vi "CRYO_MASTER_FULL_dev.vi"() -> ()   [LabVIEW 2017] (continued)
              tunnel: [w493] -> w489
              tunnel: w491 -> [w508]
              tunnel: w489 -> [w496]
              tunnel: [w495] -> w488
              tunnel: w487 -> [w494]
              frame #0 {
                n241 = property class="TabCtl (strict)"("Val(Sgnl)"=T1."DMMs" ("Value (Signaling)")) -> ()  [unwired: 2 in, 2 out]
              }
              frame #1 {
                w506 = "_" ("string")
                n242 = local read "Cycle #"() -> (w504:u32)
                n243 = call "LV_UNIXTIME.vi"("current time"=w496) -> ("date/time string"=w507:string)  [unwired: 9 in, 1 out]
                n244 = Format Value(format string="%06d", value (0)=w504) -> (output string=w503:string)  [unwired: 1 in]
                n245 = Concatenate Strings(w494, w507, w506, w503, w506, "page6.png" ("string")) -> (w501:string)
                n246 = invoke class="TabCtl (strict)" method="Get Image"(error in=errorcluster {"status"=FALSE, "code"=0, "source"=""} ("error in (no error)")) -> (error out=w497:errorcluster, "image data"=w499:T23)  [unwired: 5 in, 4 out]
                n247 = Build Path(base path=w508, name or relative path=w501) -> (appended path=w500:path)
                n248 = call <vilib>:"Write PNG File.vi"("error in (no error)"=w497, "image data"=w499, "path to PNG file"=w500) -> ("error out"=w495:errorcluster)  [unwired: 7 in, 1 out]
              }
            }
            n249 = local write "error out (frontpanel screenshots)"(w488) -> ()
          }
          frame #6 {
            n250 = flat-sequence {
              tunnel: w512 -> [w515]
              tunnel: [w515] -> w511
              tunnel: w513 -> [w530]
              tunnel: w511 -> [w518]
              tunnel: [w517] -> w510
              tunnel: w509 -> [w516]
              frame #0 {
                n251 = property class="TabCtl (strict)"("Val(Sgnl)"=T1."DIAGRAM" ("Value (Signaling)")) -> ()  [unwired: 2 in, 2 out]
              }
              frame #1 {
                w528 = "_" ("string")
                n252 = local read "Cycle #"() -> (w526:u32)
                n253 = Format Value(format string="%06d", value (0)=w526) -> (output string=w525:string)  [unwired: 1 in]
                n254 = call "LV_UNIXTIME.vi"("current time"=w518) -> ("date/time string"=w529:string)  [unwired: 9 in, 1 out]
                n255 = Concatenate Strings(w516, w529, w528, w525, w528, "page7.png" ("string")) -> (w523:string)
                n256 = invoke class="TabCtl (strict)" method="Get Image"(error in=errorcluster {"status"=FALSE, "code"=0, "source"=""} ("error in (no error)")) -> (error out=w519:errorcluster, "image data"=w521:T23)  [unwired: 5 in, 4 out]
                n257 = Build Path(base path=w530, name or relative path=w523) -> (appended path=w522:path)
                n258 = call <vilib>:"Write PNG File.vi"("error in (no error)"=w519, "image data"=w521, "path to PNG file"=w522) -> ("error out"=w517:errorcluster)  [unwired: 7 in, 1 out]
              }
            }
            n259 = local write "error out (frontpanel screenshots)"(w510) -> ()
          }
          frame #7 {
            n260 = flat-sequence {
              tunnel: w534 -> [w537]
              tunnel: [w537] -> w533
              tunnel: w535 -> [w552]
              tunnel: w533 -> [w540]
              tunnel: [w539] -> w532
              tunnel: w531 -> [w538]
              frame #0 {
                n261 = property class="TabCtl (strict)"("Val(Sgnl)"=T1."CHF" ("Value (Signaling)")) -> ()  [unwired: 2 in, 2 out]
              }
              frame #1 {
                w550 = "_" ("string")
                n262 = local read "Cycle #"() -> (w548:u32)
                n263 = Format Value(format string="%06d", value (0)=w548) -> (output string=w547:string)  [unwired: 1 in]
                n264 = call "LV_UNIXTIME.vi"("current time"=w540) -> ("date/time string"=w551:string)  [unwired: 9 in, 1 out]
                n265 = Concatenate Strings(w538, w551, w550, w547, w550, "page8.png" ("string")) -> (w545:string)
                n266 = invoke class="TabCtl (strict)" method="Get Image"(error in=errorcluster {"status"=FALSE, "code"=0, "source"=""} ("error in (no error)")) -> (error out=w541:errorcluster, "image data"=w543:T23)  [unwired: 5 in, 4 out]
                n267 = Build Path(base path=w552, name or relative path=w545) -> (appended path=w544:path)
                n268 = call <vilib>:"Write PNG File.vi"("error in (no error)"=w541, "image data"=w543, "path to PNG file"=w544) -> ("error out"=w539:errorcluster)  [unwired: 7 in, 1 out]
              }
            }
            n269 = local write "error out (frontpanel screenshots)"(w532) -> ()
          }
          frame #8 {
            n270 = flat-sequence {
              tunnel: w556 -> [w559]
              tunnel: [w559] -> w555
              tunnel: w557 -> [w574]
              tunnel: w555 -> [w562]
              tunnel: [w561] -> w554
              tunnel: w553 -> [w560]
              frame #0 {
                n271 = property class="TabCtl (strict)"("Val(Sgnl)"=T1."(Plc. hld.)" ("Value (Signaling)")) -> ()  [unwired: 2 in, 2 out]
              }
              frame #1 {
                w572 = "_" ("string")
                n272 = local read "Cycle #"() -> (w570:u32)
                n273 = Format Value(format string="%06d", value (0)=w570) -> (output string=w569:string)  [unwired: 1 in]
                n274 = call "LV_UNIXTIME.vi"("current time"=w562) -> ("date/time string"=w573:string)  [unwired: 9 in, 1 out]
                n275 = Concatenate Strings(w560, w573, w572, w569, w572, "page8.png" ("string")) -> (w567:string)
                n276 = invoke class="TabCtl (strict)" method="Get Image"(error in=errorcluster {"status"=FALSE, "code"=0, "source"=""} ("error in (no error)")) -> (error out=w563:errorcluster, "image data"=w565:T23)  [unwired: 5 in, 4 out]
                n277 = Build Path(base path=w574, name or relative path=w567) -> (appended path=w566:path)
                n278 = call <vilib>:"Write PNG File.vi"("error in (no error)"=w563, "image data"=w565, "path to PNG file"=w566) -> ("error out"=w561:errorcluster)  [unwired: 7 in, 1 out]
              }
            }
            n279 = local write "error out (frontpanel screenshots)"(w554) -> ()
          }
          frame #9 {
            n280 = local write "Frontpanel screenshots"(FALSE ("Frontpanel screenshots")) -> ()
          }
        }
        "error out (frontpanel screenshots)" <- w373
        n281 = property class="TabCtl (strict)"("Val(Sgnl)"=w371) -> ()  [unwired: 2 in, 2 out]
      }
      event "Stop Button": Value Change {
        n282 = event-data() -> ()  [unwired: 1 in, 3 out]
      }
    }
    n283 = Wait (ms)(milliseconds to wait=u32 123) -> ()  [unwired: 1 out]
  }
  n284 = while {
    stop <- w581 stop-if-true
    n285 = event shown="[5] \"Plot selecter LSI218(1)     1      2     3     4\", \"Plot selecter LSI218(2)     1      2     3     4\", \"Plot selecter (USB6210)     1      2     3     4\", \"Plot selecter LSI336       1      2     3     4\", \"Plot selecter (USB6218)     1      2     3     4\": Value Change" {
      selector: _ -> [_ _ _ _ _ _ _ _ _ _ _]
      dyn-events: _ -> [_ _ _ _ _ _ _ _ _ _ _]
      timeout: _ -> [_ _ _ _ _ _ _ _ _ _ _]
      tunnel: [_ _ _ _ _ _ _ _ _ _ TRUE] -> w581
      tunnel: [errorcluster {"status"=FALSE, "code"=0, "source"=""} ("error out") w585 _ _ _ _ w721 w738 w755 w772 errorcluster {"status"=FALSE, "code"=0, "source"=""} ("error out")] -> w577
      event Timeout {
        n286 = event-data() -> ()  [unwired: 1 in, 3 out]
      }
      event "log/linear 1": Value Change {
        n287 = event-data() -> ()  [unwired: 1 in, 6 out]
        n288 = flat-sequence {
          tunnel: [w586] -> w585
          frame #0 {
            n289 = Boolean To (0,1)(Boolean="log/linear 1") -> (0, 1=w591:i16)
            n290 = control-ref of="Graph 1"() -> (w587:refnum<vi>)
            n291 = property class="XYGraph (strict)"(reference=w587, error in=errorcluster {"status"=FALSE, "code"=0, "source"=""} ("error in (no error)"), "YScale.Mapping Mode"=w591) -> (error out=w589:errorcluster)  [unwired: 1 out]
            n292 = control-ref of="error out (USB6210)"() -> (w590:refnum<vi>)
            n293 = property class="Clust (strict)"(reference=w590, "Val(Sgnl)"=w589) -> (error out=w586:errorcluster)  [unwired: 1 in, 1 out]
          }
        }
      }
      event "log/linear 2": Value Change {
        n294 = event-data() -> ()  [unwired: 1 in, 6 out]
        n295 = flat-sequence {
          frame #0 {
            n296 = Boolean To (0,1)(Boolean="log/linear 2") -> (0, 1=w597:i16)
            n297 = control-ref of="Graph 2"() -> (w595:refnum<vi>)
            n298 = property class="XYGraph (strict)"(reference=w595, error in=errorcluster {"status"=FALSE, "code"=0, "source"=""} ("error in (no error)"), "YScale.Mapping Mode"=w597) -> (error out=w596:errorcluster)  [unwired: 1 out]
            n299 = control-ref of="error out (USB6210)"() -> (w594:refnum<vi>)
            n300 = property class="Clust (strict)"(reference=w594, "Value"=w596) -> ()  [unwired: 1 in, 2 out]
          }
        }
      }
      event "log/linear 3": Value Change {
        n301 = event-data() -> ()  [unwired: 1 in, 6 out]
        n302 = flat-sequence {
          frame #0 {
            n303 = Boolean To (0,1)(Boolean="log/linear 3") -> (0, 1=w603:i16)
            n304 = control-ref of="Graph 3"() -> (w599:refnum<vi>)
            n305 = property class="XYGraph (strict)"(reference=w599, error in=errorcluster {"status"=FALSE, "code"=0, "source"=""} ("error in (no error)"), "YScale.Mapping Mode"=w603) -> (error out=w602:errorcluster)  [unwired: 1 out]
            n306 = control-ref of="error out (USB6210)"() -> (w601:refnum<vi>)
            n307 = property class="Clust (strict)"(reference=w601, "Value"=w602) -> ()  [unwired: 1 in, 2 out]
          }
        }
      }
      event "log/linear 4": Value Change {
        n308 = event-data() -> ()  [unwired: 1 in, 6 out]
        n309 = flat-sequence {
          frame #0 {
            n310 = Boolean To (0,1)(Boolean="log/linear 4") -> (0, 1=w609:i16)
            n311 = control-ref of="Graph 4"() -> (w605:refnum<vi>)
            n312 = property class="XYGraph (strict)"(reference=w605, error in=errorcluster {"status"=FALSE, "code"=0, "source"=""} ("error in (no error)"), "YScale.Mapping Mode"=w609) -> (error out=w608:errorcluster)  [unwired: 1 out]
            n313 = control-ref of="error out (USB6210)"() -> (w607:refnum<vi>)
            n314 = property class="Clust (strict)"(reference=w607, "Value"=w608) -> ()  [unwired: 1 in, 2 out]
          }
        }
      }
      event "Plot selecter LSI218(1)\n    1      2     3     4", "Plot selecter LSI218(2)\n    1      2     3     4", "Plot selecter (USB6210)\n    1      2     3     4", "Plot selecter LSI336 \n     1      2     3     4", "Plot selecter (USB6218)\n    1      2     3     4": Value Change {
        n315 = event-data() -> ()  [unwired: 1 in, 6 out]
        n316 = local read "Labels (HP34401 LM)"() -> (w616:string[])
        n317 = call "BuildPlotLegends.vi"("Plot selecter \n    1      2     3     4"="Plot selecter (HP34401A)\n    1      2     3     4", "AllLabels"=w616) -> ("Series 4"=w611:string[], "Series 3"=w612:string[], "Series 2"=w613:string[], "Series 1"=w614:string[])  [unwired: 6 in]
        n318 = local read "All Labels (USB6210)"() -> (w633:string[])
        n319 = local read "All Labels (USB6218)"() -> (w622:string[])
        n320 = local read "Labels LSI218 (1)"() -> (w635:string[])
        n321 = local read "Labels LSI218 (2)"() -> (w636:string[])
        n322 = local read "Labels LSI336"() -> (w628:string[])
        n323 = call "BuildPlotLegends_LSI218.vi"("Plot selecter (2)\n    1      2     3     5"="Plot selecter LSI218(2)\n    1      2     3     4", "Plot selecter (1)\n    1      2     3     4"="Plot selecter LSI218(1)\n    1      2     3     4", "Labels (2)"=w636, "Labels (1)"=w635) -> ("Series 4"=w646:string[], "Series 3"=w644:string[], "Series 2"=w642:string[], "Series 1"=w640:string[])  [unwired: 4 in]
        n324 = call "BuildPlotLegends.vi"("Plot selecter \n    1      2     3     4"="Plot selecter (USB6210)\n    1      2     3     4", "AllLabels"=w633) -> ("Series 4"=w645:string[], "Series 3"=w643:string[], "Series 2"=w641:string[], "Series 1"=w639:string[])  [unwired: 6 in]
        n325 = call "BuildPlotLegends.vi"("Plot selecter \n    1      2     3     4"="Plot selecter LSI336 \n     1      2     3     4", "AllLabels"=w628) -> ("Series 4"=w623:string[], "Series 3"=w624:string[], "Series 2"=w625:string[], "Series 1"=w626:string[])  [unwired: 6 in]
        n326 = call "BuildPlotLegends.vi"("Plot selecter \n    1      2     3     4"="Plot selecter (USB6218)\n    1      2     3     4", "AllLabels"=w622) -> ("Series 4"=w618:string[], "Series 3"=w617:string[], "Series 2"=w619:string[], "Series 1"=w620:string[])  [unwired: 6 in]
        n327 = Build Array (concatenate)(w641, w642, w625, w619, w613) -> (w630:string[])
        "Series 2" <- w630
        n328 = Build Array (concatenate)(w643, w644, w624, w617, w612) -> (w631:string[])
        "Series 3" <- w631
        n329 = Build Array (concatenate)(w645, w646, w623, w618, w611) -> (w632:string[])
        "Series 4" <- w632
        n330 = Build Array (concatenate)(w639, w640, w626, w620, w614) -> (w629:string[])
        "Series 1" <- w629
        n331 = stacked-sequence {
          tunnel: [w656 _ _ _] -> w650
          tunnel: [_ w674 _ _] -> w651
          tunnel: [_ _ w691 _] -> w649
          tunnel: [_ _ _ w708] -> w648
          tunnel: w629 -> [w654 _ _ _]
          tunnel: w630 -> [_ w672 _ _]
          tunnel: w631 -> [_ _ w689 _]
          tunnel: w632 -> [_ _ _ w706]
          frame #0 {
            n332 = Array Size(array=w654) -> (size(s)=w658:i32)
            n333 = control-ref of="Graph 1"() -> (w652:refnum<vi>)
            n334 = property class="XYGraph (strict)"(reference=w652) -> ("LegNumRows"=w653:u32)  [unwired: 1 in, 2 out]
            n335 = for {
              N: w653 -> [_]
              tunnel: w652 -> [w667]
              shift-right: [w665] -> w657
              shift-left: errorcluster {"status"=FALSE, "code"=0, "source"=""} ("error in (no error)") -> [w666]
              i -> [w669]
              n336 = property class="XYGraph (strict)"(reference=w667, error in=w666, "Active Plot"=w669, "Plot.Plot Name"="") -> (error out=w665:errorcluster)  [unwired: 1 out]
            }
            n337 = for {
              N: w658 -> [_]
              tunnel: w652 -> [w663]
              shift-right: [w661] -> w656
              shift-left: w657 -> [w662]
              tunnel: w654 -> [w660] mode=indexing
              i -> [w664]
              n338 = property class="XYGraph (strict)"(reference=w663, error in=w662, "Active Plot"=w664, "Plot.Plot Name"=w660, "Plot.Visible?"=TRUE ("Plot.Visible")) -> (error out=w661:errorcluster)  [unwired: 1 out]
            }
          }
          frame #1 {
            n339 = Array Size(array=w672) -> (size(s)=w676:i32)
            n340 = control-ref of="Graph 2"() -> (w671:refnum<vi>)
            n341 = property class="XYGraph (strict)"(reference=w671) -> ("LegNumRows"=w670:u32)  [unwired: 1 in, 2 out]
            n342 = for {
              N: w670 -> [_]
              shift-right: [w683] -> w675
              shift-left: errorcluster {"status"=FALSE, "code"=0, "source"=""} ("error in (no error)") -> [w684]
              tunnel: w671 -> [w682]
              i -> [w686]
              n343 = property class="XYGraph (strict)"(reference=w682, error in=w684, "Active Plot"=w686, "Plot.Plot Name"="") -> (error out=w683:errorcluster)  [unwired: 1 out]
            }
            n344 = for {
              N: w676 -> [_]
              shift-right: [w679] -> w674
              shift-left: w675 -> [w680]
              tunnel: w672 -> [w678] mode=indexing
              tunnel: w671 -> [w677]
              i -> [w681]
              n345 = property class="XYGraph (strict)"(reference=w677, error in=w680, "Active Plot"=w681, "Plot.Plot Name"=w678) -> (error out=w679:errorcluster)  [unwired: 1 out]
            }
          }
          frame #2 {
            n346 = Array Size(array=w689) -> (size(s)=w693:i32)
            n347 = control-ref of="Graph 3"() -> (w687:refnum<vi>)
            n348 = property class="XYGraph (strict)"(reference=w687) -> ("LegNumRows"=w688:u32)  [unwired: 1 in, 2 out]
            n349 = for {
              N: w688 -> [_]
              tunnel: w687 -> [w701]
              shift-right: [w699] -> w692
              shift-left: errorcluster {"status"=FALSE, "code"=0, "source"=""} ("error in (no error)") -> [w700]
              i -> [w703]
              n350 = property class="XYGraph (strict)"(reference=w701, error in=w700, "Active Plot"=w703, "Plot.Plot Name"="") -> (error out=w699:errorcluster)  [unwired: 1 out]
            }
            n351 = for {
              N: w693 -> [_]
              tunnel: w687 -> [w697]
              shift-right: [w695] -> w691
              shift-left: w692 -> [w696]
              tunnel: w689 -> [w694] mode=indexing
              i -> [w698]
              n352 = property class="XYGraph (strict)"(reference=w697, error in=w696, "Active Plot"=w698, "Plot.Plot Name"=w694) -> (error out=w695:errorcluster)  [unwired: 1 out]
            }
          }
          frame #3 {
            n353 = Array Size(array=w706) -> (size(s)=w710:i32)
            n354 = control-ref of="Graph 4"() -> (w704:refnum<vi>)
            n355 = property class="XYGraph (strict)"(reference=w704) -> ("LegNumRows"=w705:u32)  [unwired: 1 in, 2 out]
            n356 = for {
              N: w705 -> [_]
              tunnel: w704 -> [w718]
              shift-right: [w716] -> w709
              shift-left: errorcluster {"status"=FALSE, "code"=0, "source"=""} ("error in (no error)") -> [w717]
              i -> [w720]
              n357 = property class="XYGraph (strict)"(reference=w718, error in=w717, "Active Plot"=w720, "Plot.Plot Name"="") -> (error out=w716:errorcluster)  [unwired: 1 out]
            }
            n358 = for {
              N: w710 -> [_]
              tunnel: w704 -> [w714]
              shift-right: [w712] -> w708
              shift-left: w709 -> [w713]
              tunnel: w706 -> [w711] mode=indexing
              i -> [w715]
              n359 = property class="XYGraph (strict)"(reference=w714, error in=w713, "Active Plot"=w715, "Plot.Plot Name"=w711) -> (error out=w712:errorcluster)  [unwired: 1 out]
            }
          }
        }
        n360 = Merge Errors(w650, w651, w649, w648) -> (→"Plot errors":errorcluster)
      }
      event "Take Screenshot! 1": Value Change {
        n361 = event-data() -> ()  [unwired: 1 in, 6 out]
        n362 = flat-sequence {
          tunnel: [w722] -> w721
          frame #0 {
            n363 = flat-sequence {
              tunnel: [w723] -> w722
              frame #0 {
                w732 = "_" ("string")
                n364 = Get Date/Time In Seconds() -> (seconds since 1Jan1904=w729:timestamp)
                n365 = local read "RUN Identifier"() -> (w734:string)
                n366 = call "LV_UNIXTIME.vi"("current time"=w729) -> ("date/time string"=w733:string)  [unwired: 9 in, 1 out]
                n367 = control-ref of="Graph 1"() -> (w728:refnum<vi>)
                n368 = Concatenate Strings(w734, w732, w733, w732, "FIle suffix 1", ".png" ("string")) -> (w736:string)
                n369 = local read "Base Path"() -> (w735:path)
                n370 = invoke class="XYGraph (strict)" method="Get Image"(reference=w728, error in=errorcluster {"status"=FALSE, "code"=0, "source"=""} ("error in (no error)")) -> (error out=w724:errorcluster, "image data"=w727:T23)  [unwired: 4 in, 4 out]
                n371 = Build Path(base path=w735, name or relative path=w736) -> (appended path=w726:path)
                n372 = call <vilib>:"Write PNG File.vi"("error in (no error)"=w724, "image data"=w727, "path to PNG file"=w726) -> ("error out"=w723:errorcluster)  [unwired: 7 in, 1 out]
              }
              frame #1 {
                n373 = local write "Take Screenshot! 1"(FALSE ("Take Screenshot! 1")) -> ()
              }
            }
          }
        }
      }
      event "Take Screenshot! 2": Value Change {
        n374 = event-data() -> ()  [unwired: 1 in, 6 out]
        n375 = flat-sequence {
          tunnel: [w739] -> w738
          frame #0 {
            n376 = flat-sequence {
              tunnel: [w745] -> w739
              frame #0 {
                w749 = "_" ("string")
                n377 = Get Date/Time In Seconds() -> (seconds since 1Jan1904=w746:timestamp)
                n378 = local read "RUN Identifier"() -> (w751:string)
                n379 = call "LV_UNIXTIME.vi"("current time"=w746) -> ("date/time string"=w750:string)  [unwired: 9 in, 1 out]
                n380 = control-ref of="Graph 2"() -> (w740:refnum<vi>)
                n381 = Concatenate Strings(w751, w749, w750, w749, "FIle suffix 2", ".png" ("string")) -> (w753:string)
                n382 = local read "Base Path"() -> (w752:path)
                n383 = invoke class="XYGraph (strict)" method="Get Image"(reference=w740, error in=errorcluster {"status"=FALSE, "code"=0, "source"=""} ("error in (no error)")) -> (error out=w744:errorcluster, "image data"=w742:T23)  [unwired: 4 in, 4 out]
                n384 = Build Path(base path=w752, name or relative path=w753) -> (appended path=w741:path)
                n385 = call <vilib>:"Write PNG File.vi"("error in (no error)"=w744, "image data"=w742, "path to PNG file"=w741) -> ("error out"=w745:errorcluster)  [unwired: 7 in, 1 out]
              }
              frame #1 {
                n386 = local write "Take Screenshot! 2"(FALSE ("Take Screenshot! 1")) -> ()
              }
            }
          }
        }
      }
      event "Take Screenshot! 3": Value Change {
        n387 = event-data() -> ()  [unwired: 1 in, 6 out]
        n388 = flat-sequence {
          tunnel: [w756] -> w755
          frame #0 {
            n389 = flat-sequence {
              tunnel: [w758] -> w756
              frame #0 {
                w766 = "_" ("string")
                n390 = Get Date/Time In Seconds() -> (seconds since 1Jan1904=w764:timestamp)
                n391 = local read "RUN Identifier"() -> (w768:string)
                n392 = call "LV_UNIXTIME.vi"("current time"=w764) -> ("date/time string"=w767:string)  [unwired: 9 in, 1 out]
                n393 = control-ref of="Graph 3"() -> (w761:refnum<vi>)
                n394 = Concatenate Strings(w768, w766, w767, w766, "FIle suffix 3", ".png" ("string")) -> (w770:string)
                n395 = local read "Base Path"() -> (w769:path)
                n396 = invoke class="XYGraph (strict)" method="Get Image"(reference=w761, error in=errorcluster {"status"=FALSE, "code"=0, "source"=""} ("error in (no error)")) -> (error out=w759:errorcluster, "image data"=w757:T23)  [unwired: 4 in, 4 out]
                n397 = Build Path(base path=w769, name or relative path=w770) -> (appended path=w762:path)
                n398 = call <vilib>:"Write PNG File.vi"("error in (no error)"=w759, "image data"=w757, "path to PNG file"=w762) -> ("error out"=w758:errorcluster)  [unwired: 7 in, 1 out]
              }
              frame #1 {
                n399 = local write "Take Screenshot! 3"(FALSE ("Take Screenshot! 1")) -> ()
              }
            }
          }
        }
      }
      event "Take Screenshot! 4": Value Change {
        n400 = event-data() -> ()  [unwired: 1 in, 6 out]
        n401 = flat-sequence {
          tunnel: [w773] -> w772
          frame #0 {
            n402 = flat-sequence {
              tunnel: [w776] -> w773
              frame #0 {
                w783 = "_" ("string")
                n403 = Get Date/Time In Seconds() -> (seconds since 1Jan1904=w781:timestamp)
                n404 = local read "RUN Identifier"() -> (w785:string)
                n405 = call "LV_UNIXTIME.vi"("current time"=w781) -> ("date/time string"=w784:string)  [unwired: 9 in, 1 out]
                n406 = control-ref of="Graph 4"() -> (w777:refnum<vi>)
                n407 = Concatenate Strings(w785, w783, w784, w783, "FIle suffix 4", ".png" ("string")) -> (w787:string)
                n408 = local read "Base Path"() -> (w786:path)
                n409 = invoke class="XYGraph (strict)" method="Get Image"(reference=w777, error in=errorcluster {"status"=FALSE, "code"=0, "source"=""} ("error in (no error)")) -> (error out=w774:errorcluster, "image data"=w778:T23)  [unwired: 4 in, 4 out]
                n410 = Build Path(base path=w786, name or relative path=w787) -> (appended path=w779:path)
                n411 = call <vilib>:"Write PNG File.vi"("error in (no error)"=w774, "image data"=w778, "path to PNG file"=w779) -> ("error out"=w776:errorcluster)  [unwired: 7 in, 1 out]
              }
              frame #1 {
                n412 = local write "Take Screenshot! 4"(FALSE ("Take Screenshot! 1")) -> ()
              }
            }
          }
        }
      }
      event "Stop Button": Value Change {
        n413 = event-data() -> ()  [unwired: 1 in, 6 out]
      }
    }
    "error out (graph operations)" <- w577
    n414 = local write "Take Screenshot! 1"(FALSE ("Take Screenshot! 1")) -> ()
    n415 = local write "Take Screenshot! 2"(FALSE ("Take Screenshot! 1")) -> ()
    n416 = Wait (ms)(milliseconds to wait=u32 1000) -> ()  [unwired: 1 out]
    n417 = local write "Take Screenshot! 3"(FALSE ("Take Screenshot! 1")) -> ()
    n418 = local write "Take Screenshot! 4"(FALSE ("Take Screenshot! 1")) -> ()
  }
  n419 = while {
    i -> [w795]
    stop <- w792 stop-if-true
    n420 = Equal?(x=w795, y=0) -> (x = y?=w793:bool)
    n421 = case shown="True" w793 {
      frame False {
      }
      frame True {
        n422 = property on="Agilent\nIntialized?" class="Bool (strict)"("Val(Sgnl)"=FALSE ("Value (Signaling)")) -> ()  [unwired: 2 in, 2 out]
      }
    }
    n423 = Wait (ms)(milliseconds to wait=u32 123) -> ()  [unwired: 1 out]
    n424 = event shown="[4] \"V_lim_up (V)\", \"V_lim_low (V)\": Value Change" {
      selector: _ -> [_ _ _ _ _]
      dyn-events: _ -> [_ _ _ _ _]
      timeout: _ -> [_ _ _ _ _]
      tunnel: [FALSE ("Value (Signaling)") TRUE ("Value (Signaling)") _ _ _] -> w792
      tunnel: "VISA (Agilent 34402)" -> [_ _ w801 w804 _]
      event Timeout {
        n425 = event-data() -> ()  [unwired: 1 in, 3 out]
      }
      event "Stop Button": Value Change {
        n426 = event-data() -> ()  [unwired: 1 in, 3 out]
      }
      event "Initialize (Agilent)": Value Change {
        n427 = event-data() -> ()  [unwired: 1 in, 3 out]
        n428 = property on="Agilent\nIntialized?" class="Bool (strict)"("Val(Sgnl)"=TRUE ("Value (Signaling)")) -> ()  [unwired: 2 in, 2 out]
        n429 = call "Initialize.vi"("error in (no error)"=errorcluster {"status"=FALSE, "code"=0, "source"=""}, "VISA resource name"=w801) -> ("error out"=→"error out (Agilent)":errorcluster)  [unwired: 8 in, 1 out]
      }
      event "OUTPUT \nKenwood", "Kenwood set V (V)": Value Change {
        n430 = local read "Agilent\nIntialized?"() -> (w803:bool)
        n431 = event-data() -> ()  [unwired: 1 in, 3 out]
        n432 = case shown="True" w803 {
          tunnel: w804 -> [_ w810]
          frame False {
          }
          frame True {
            w812 = u16 0 items=["DC", "Sine", "Square", "Triangle", "Ramp", "Pulse", "Noise", "Sinc", "Negative Ramp", "Exponential Rise", "Exponential Fall", "Cardiac"] ("Waveform Function (1: Sine)")
            n433 = xnode "Formula"("X1"="Kenwood set V (V)") -> ("Result"=w805:dbl)  [unwired: 1 in, 1 out]
            n434 = call "Configure Standard Waveform.vi"("DC Offset (0.00 V)"=w805, "Frequency (1000 Hz)"=1.0, "error in (no error)"=errorcluster {"status"=FALSE, "code"=0, "source"=""}, "Amplitude (1)"=1.0, "Waveform Function (1: Sine)"=w812, "VISA resource name"=w810) -> ("error out"=w814:errorcluster, "VISA resource name out"=w815:refnum<visa-resource-name>)  [unwired: 4 in]
            n435 = call "Enable Output.vi"("error in (no error)"=w814, "Enable Output  (T: Enable)"="OUTPUT \nKenwood", "VISA resource name"=w815) -> ("error out"=w808:errorcluster)  [unwired: 7 in, 1 out]
            n436 = local write "error out (Agilent)"(w808) -> ()
          }
        }
      }
      event "V_lim_up (V)", "V_lim_low (V)": Value Change {
        n437 = event-data() -> ()  [unwired: 1 in, 3 out]
        n438 = property on="Kenwood set V (V)" class="DigNum (strict)"("Minimum"="V_lim_low (V)", "Maximum"="V_lim_up (V)") -> ()  [unwired: 2 in, 2 out]
      }
    }
  }
  n439 = while {
    stop <- w827 stop-if-true
    n440 = Wait (ms)(milliseconds to wait=u32 101) -> ()  [unwired: 1 out]
    n441 = event shown="[2] Timeout" {
      selector: _ -> [_ _ _]
      dyn-events: _ -> [_ _ _]
      timeout: _ -> [_ _ _]
      tunnel: [FALSE TRUE FALSE] -> w827
      event "Initialize (DMMs)": Value Change {
        w830 = T4 [] ("Value (Signaling)")
        n442 = event-data() -> ()  [unwired: 1 in, 3 out]
        n443 = property on="Graph DMMs 1" class="XYGraph (strict)"("Val(Sgnl)"=w830) -> ()  [unwired: 2 in, 2 out]
        n444 = property on="Graph DMMs 2" class="XYGraph (strict)"("Val(Sgnl)"=w830) -> ()  [unwired: 2 in, 2 out]
      }
      event "Stop Button": Value Change {
        n445 = event-data() -> ()  [unwired: 1 in, 3 out]
      }
      event Timeout {
        n446 = event-data() -> ()  [unwired: 1 in, 3 out]
      }
    }
  }
  n447 = Obtain Notifier(name (unnamed)="stop notifier", notification data type=w17, create if not found? (T)=w17, error in (no error)=errorcluster {"status"=FALSE, "code"=0, "source"=""}) -> (notifier out=w5:refnum<notifier>, error out=w4:errorcluster)  [unwired: 1 out]
  n448 = while {
    shift-right: [w943] -> w40
    shift-left: refnum<class "USBData.lvclass"> refnum ("USBData.lvclass") -> [w946]
    shift-right: [w939] -> w39
    shift-left: w6 -> [w945]
    tunnel: "Base Path" -> [w845]
    shift-right: [w921] -> w34
    shift-left: errorcluster {"status"=FALSE, "code"=0, "source"=""} ("error in (no error)") -> [w937]
    shift-right: [w922] -> w35
    shift-left: refnum<class "LSI218Data.lvclass"> refnum ("LSI218Data.lvclass") -> [w936]
    shift-right: [w909] -> w31
    shift-left: refnum<class "LSI336Data.lvclass"> refnum ("LSI336Data.lvclass") -> [w918]
    shift-right: [w908] -> w30
    shift-left: w21 -> [w917]
    shift-right: [w897] -> _
    shift-left: w6 -> [w898]
    shift-right: [w887] -> w25
    shift-left: refnum<class "USBData.lvclass"> refnum ("USBData.lvclass") -> [w895]
    shift-right: [w886] -> w24
    shift-left: errorcluster {"status"=FALSE, "code"=0, "source"=""} ("error in (no error)") -> [w894]
    shift-right: [w883] -> _
    shift-left: w21 -> [w882]
    tunnel: w5 -> [w853]
    tunnel: w4 -> [w852]
    tunnel: [w850] -> w13
    tunnel: [w849] -> w12
    shift-right: [w846] -> _
    shift-left: refnum<class "LMData.lvclass"> refnum ("LMData in") -> [w847]
    shift-right: [w843] -> _
    shift-left: errorcluster {"status"=FALSE, "code"=0, "source"=""} ("error in (no error)") -> [w844]
    i -> [w842]
    stop <- "Stop Button" stop-if-true
    w838 = T25 [] ("appended array")
    w904 = u32 24 ("Number of Rows")
    w914 = T25 [] ("appended array")
    w931 = T25 [] ("appended array")
    n449 = local read "LSI218Settings(A-F)"() -> (w874:T3)
    n450 = control-ref of="Plot selecter LSI218(2)\n    1      2     3     4"() -> (w902:refnum<vi>)
    n451 = control-ref of="Plot selecter LSI218(1)\n    1      2     3     4"() -> (w903:refnum<vi>)
    n452 = control-ref of="Plot selecter LSI336 \n     1      2     3     4"() -> (w901:refnum<vi>)
    n453 = property on="Property Node" class="Arr (strict)"(reference=w902, "Number of Rows"=w904) -> ()  [unwired: 1 in, 2 out]
    n454 = property on="Property Node" class="Arr (strict)"(reference=w903, "Number of Rows"=w904) -> ()  [unwired: 1 in, 2 out]
    n455 = local read "LSI336Settings(X,Y)"() -> (w872:T3)
    n456 = Array Size(array=w874) -> (size(s)=w873:i32)
    n457 = property on="Property Node" class="Arr (strict)"(reference=w901, "Number of Rows"=u32 8) -> ()  [unwired: 1 in, 2 out]
    n458 = Multiply(x="Measurement Interval (s)", y=u32 1000) -> (x*y=w940:dbl)
    n459 = Wait (ms)(milliseconds to wait=w940) -> ()  [unwired: 1 out]
    n460 = for {
      N: w873 -> [_]
      tunnel: w874 -> [w1032] mode=indexing
      tunnel: [w1031] -> w870 mode=concatenating
      n461 = Unbundle By Name(w1032) -> ("SensorLocations"=w1031:T18)
    }
    n462 = for {
      tunnel: w872 -> [w1030] mode=indexing
      tunnel: [w1029] -> w871 mode=concatenating
      n463 = Unbundle By Name(w1030) -> ("SensorLocations"=w1029:T18)
    }
    n464 = Quotient & Remainder(x=w842, y="Screenshots interval") -> (x-y*floor(x/y)=w858:i64)  [unwired: 1 out]
    n465 = Equal?(x=w842, y=0) -> (x = y?=w848:bool)
    n466 = case shown="True" w848 {
      tunnel: w946 -> [w2097 w2120]
      tunnel: w945 -> [w2091 w2118]
      tunnel: w842 -> [w2082 _]
      tunnel: [w2089 w2115] -> w939
      tunnel: [w2086 w2114] -> w896
      tunnel: [w2087 w2113] -> w943
      tunnel: [w2077 w2108] -> w944
      tunnel: w845 -> [_ w2107]
      tunnel: [w2076 w2104] -> w879
      frame False {
        n467 = call-dynamic "USBData_measure.vi"("USBData in"=w2097, "DAQ sample #"=i64 5, "DAQ timeout"=100.0 ("DAQ timeout (def: 100)"), "MeasurementIndex"=w2082, "error in (no error)"=w2091, "save every ... measurements"="Record interval") -> ("USBData out"=w2096:refnum<class "USBData.lvclass">, "TimeMeasuremeent"=w2093:timestamp, "Status"=→"USB6210 Status":T6, "LastDataAcquired"=w2078:dbl[], "error out"=w2092:errorcluster)  [unwired: 3 in, 2 out]
        "Time of Last Measurement (USB6210)" <- w2093
        "Last Vol\n(USB6210)" <- w2078
        n468 = call-dynamic "USBData_convert.vi"("Save every ... measurements"="Record interval", "MeasurementIndex"=w2082, "error in (no error)"=w2092, "LastDataAcquired"=w2078, "TimeMeasuremeent"=w2093, "USBData in"=w2096) -> ("error out"=w2090:errorcluster, "LeakDet_FULL"=w2085:dbl, "LastDataConverted"=w2079:dbl[], "USBData out"=w2088:refnum<class "USBData.lvclass">)  [unwired: 2 in]
        n469 = call "USBData_read.vi"("USBData in"=w2088, "error in (no error)"=w2090) -> ("Status"=w2080:T6, "USBData out"=w2087:refnum<class "USBData.lvclass">, "Data"=w2086:T26, "Basic"=w2077:T27, "error out"=w2089:errorcluster)  [unwired: 2 in, 2 out]
        n470 = local write "USB6210 Status"(w2080) -> ()
        n471 = Unbundle By Name(w2077) -> ("ReadLeakDet?"=w2084:bool)
        n472 = Unbundle By Name(w2077) -> ("Labels"=w2076:string[])
        n473 = case shown="False" w2084 {
          tunnel: w2079 -> [w2098 w2101]
          tunnel: w2085 -> [_ w2100]
          tunnel: [w2098 w2099] -> w2083
          frame False {
          }
          frame True {
            n474 = Build Array (concatenate)(w2101, w2100) -> (w2099:dbl[])
          }
        }
        "Last Data \n(USB6210)" <- w2083
      }
      frame True {
        n475 = local read "RUN Identifier"() -> (w2102:string)
        n476 = call-dynamic "USBData_initialize.vi"("USBData in"=w2120, "SeriesSetting"="USB6210 Config", "BasePath"=w2107, "RunIdentifier"=w2102, "FileName"="InstName (USB6210)", "error in (no error)"=w2118) -> ("Status"=w2103:T6, "USBData out"=w2116:refnum<class "USBData.lvclass">, "error out"=w2117:errorcluster)  [unwired: 5 in, 2 out]
        n477 = local write "USB6210 Status"(w2103) -> ()
        n478 = call "USBData_read.vi"("USBData in"=w2116, "error in (no error)"=w2117) -> ("Status"=w2106:T6, "USBData out"=w2113:refnum<class "USBData.lvclass">, "Data"=w2114:T26, "Basic"=w2108:T27, "error out"=w2115:errorcluster)  [unwired: 2 in, 2 out]
        n479 = local write "USB6210 Status"(w2106) -> ()
        n480 = Unbundle By Name(w2108) -> ("ReadLeakDet?"=w2112:bool, "Labels"=w2104:string[])
        n481 = Array Size(array=w2104) -> (size(s)=w2111:i32)
        n482 = case shown="True" w2112 {
          tunnel: w2111 -> [w2121 w2123]
          tunnel: [w2121 w2122] -> w2109
          frame False {
          }
          frame True {
            n483 = Add(x=w2123, y=1) -> (x+y=w2122:i32)
          }
        }
        n484 = Initialize Array(TRUE ("Activate 2"), w2109) -> ()  [unwired: 1 out]
      }
    }
    "error out (USB6210)" <- w939
    n485 = case shown="False" w848 {
      tunnel: [w1613 w1640] -> w886
      tunnel: [w1610 w1639] -> w893
      tunnel: [w1611 w1638] -> w887
      tunnel: [w1602 w1633] -> w892
      tunnel: [w1601 w1631] -> _
      tunnel: w895 -> [w1600 w1629]
      tunnel: w845 -> [_ w1628]
      tunnel: w894 -> [w1599 w1627]
      tunnel: w842 -> [w1598 _]
      frame False {
        n486 = local read "Record interval"() -> (w1597:i64)
        n487 = call-dynamic "USBData_measure.vi"("USBData in"=w1600, "DAQ sample #"=i64 5, "DAQ timeout"=100.0 ("DAQ timeout (def: 100)"), "MeasurementIndex"=w1598, "error in (no error)"=w1599, "save every ... measurements"=w1597) -> ("USBData out"=w1619:refnum<class "USBData.lvclass">, "TimeMeasuremeent"=w1616:timestamp, "Status"=→"USB6218 Status":T6, "LastDataAcquired"=w1603:dbl[], "error out"=w1615:errorcluster)  [unwired: 3 in, 2 out]
        "Time of Last Measurement (USB6218)" <- w1616
        "Last Vol \n(USB6218)" <- w1603
        n488 = call-dynamic "USBData_convert.vi"("Save every ... measurements"=w1597, "MeasurementIndex"=w1598, "error in (no error)"=w1615, "LastDataAcquired"=w1603, "TimeMeasuremeent"=w1616, "USBData in"=w1619) -> ("error out"=w1614:errorcluster, "LeakDet_FULL"=w1609:dbl, "LastDataConverted"=w1604:dbl[], "USBData out"=w1612:refnum<class "USBData.lvclass">)  [unwired: 2 in]
        n489 = call "USBData_read.vi"("USBData in"=w1612, "error in (no error)"=w1614) -> ("Status"=w1605:T6, "USBData out"=w1611:refnum<class "USBData.lvclass">, "Data"=w1610:T26, "Basic"=w1602:T27, "error out"=w1613:errorcluster)  [unwired: 2 in, 2 out]
        n490 = local write "USB6218 Status"(w1605) -> ()
        n491 = Unbundle By Name(w1602) -> ("ReadLeakDet?"=w1608:bool)
        n492 = Unbundle By Name(w1602) -> ("Labels"=w1601:string[])
        n493 = case shown="True" w1608 {
          tunnel: w1604 -> [w1620 w1623]
          tunnel: w1609 -> [_ w1622]
          tunnel: [w1620 w1621] -> w1607
          frame False {
          }
          frame True {
            n494 = Build Array (concatenate)(w1623, w1622) -> (w1621:dbl[])
          }
        }
        "Last Data \n(USB6218)" <- w1607
      }
      frame True {
        n495 = local read "RUN Identifier"() -> (w1624:string)
        n496 = call-dynamic "USBData_initialize.vi"("USBData in"=w1629, "SeriesSetting"="USB6218 Config", "BasePath"=w1628, "RunIdentifier"=w1624, "FileName"="InstName (USB6218)", "error in (no error)"=w1627) -> ("Status"=w1625:T6, "USBData out"=w1641:refnum<class "USBData.lvclass">, "error out"=w1642:errorcluster)  [unwired: 5 in, 2 out]
        n497 = local write "USB6218 Status"(w1625) -> ()
        n498 = call "USBData_read.vi"("USBData in"=w1641, "error in (no error)"=w1642) -> ("Status"=w1632:T6, "USBData out"=w1638:refnum<class "USBData.lvclass">, "Data"=w1639:T26, "Basic"=w1633:T27, "error out"=w1640:errorcluster)  [unwired: 2 in, 2 out]
        n499 = local write "USB6218 Status"(w1632) -> ()
        n500 = Unbundle By Name(w1633) -> ("ReadLeakDet?"=w1637:bool, "Labels"=w1631:string[])
        n501 = Array Size(array=w1631) -> (size(s)=w1636:i32)
        n502 = case shown="True" w1637 {
          tunnel: w1636 -> [w1643 w1645]
          tunnel: [w1643 w1644] -> w1634
          frame False {
          }
          frame True {
            n503 = Add(x=w1645, y=1) -> (x+y=w1644:i32)
          }
        }
        n504 = Initialize Array(TRUE ("Activate 2"), w1634) -> ()  [unwired: 1 out]
      }
    }
    "error out (USB6218)" <- w886
    n505 = case shown="True" w848 {
      frame False {
      }
      frame True {
        n506 = local read "RUN label"() -> (w1023:string)
        n507 = Get Date/Time In Seconds() -> (seconds since 1Jan1904=w1027:timestamp)
        n508 = call "LV_UNIXTIME.vi"("current time"=w1027) -> ("date/time string"=w1026:string)  [unwired: 9 in, 1 out]
        n509 = Concatenate Strings(w1026, "_" ("string"), w1023) -> (→"RUN Identifier" →"RUN Identifier 2" →"RUN Identifier 3" →"RUN Identifier 4" →"RUN Identifier 5" →"RUN Identifier 6" →"RUN Identifier 7":string)
      }
    }
    n510 = Equal?(x=w858, y=i64 0) -> (x = y?=w855:bool)
    n511 = local read "LastData (LSI218)"() -> (w868:dbl[])
    n512 = local read "Last Data \nLSI336"() -> (w867:dbl[])
    n513 = And(x="Analog Out ON?", y=w848) -> (x .and. y?=w884:bool)
    n514 = And(x=w855, y="Automatic \nScreenshots?") -> (x .and. y?=w854:bool)
    n515 = Build Array (concatenate)(w868, w867) -> (w866:dbl[])
    "AllTemperatures" <- w866
    n516 = Build Array (concatenate)(w870, w871) -> (w869:T18)
    "TempSensorsLocations" <- w869
    n517 = case shown="True" w884 {
      tunnel: w845 -> [_ w1416]
      tunnel: [w1392 w1407] -> w883
      tunnel: w882 -> [w1392 w1406]
      frame False {
      }
      frame True {
        w1399 = "_raw" ("string")
        w1423 = 10.0 ("V_lim_max")
        w1422 = 0.0 ("V_lim_min")
        w1421 = -1 items=["Default"=-1, "RSE"=10083, "Differential"=10106, "Pseudodifferential"=12529] ("output terminal configuration")
        w1420 = 10348 items=["Volts"=10348, "From Custom Scale"=10065] ("units")
        n518 = local read "RUN Identifier"() -> (w1405:string)
        n519 = Concatenate Strings(w1405, "_AO" ("string")) -> (w1425:string)
        n520 = Concatenate Strings(w1405, "_", "USB_AOUT.csv" ("string")) -> (w1417:string)
        n521 = Array To Cluster(array="AOUT Labels") -> (cluster=w1403:T28)
        n522 = Unbundle By Name(w1403) -> ("AOUT Labels[0]"=w1402:string, "AOUT Labels[1]"=w1400:string)
        n523 = Build Path(base path=w1416, name or relative path=w1417) -> (appended path=w1413:path)
        n524 = Concatenate Strings(w1402, w1399) -> (w1401:string)
        n525 = Concatenate Strings(w1400, w1399) -> (w1398:string)
        n526 = Open/Create/Replace File(file path (use dialog)=w1413, operation (0:open)=T24."open or create") -> (refnum out=w1411:refnum<file>)  [unwired: 4 in, 2 out]
        n527 = Build Array(w1402, w1400, w1401, w1398) -> (w1409:string[])
        n528 = call "FileIntialize.vi"("Error In"=w1406, "Labels"=w1409, "refnum in"=w1411) -> ("Error Out"=w1408:errorcluster, "File Refnum"=→"File Refn USB AO":refnum<file>)  [unwired: 7 in]
        n529 = call <vilib>:"DAQmx Create Task.vi"("new task name"=w1425, "auto cleanup"=FALSE, "error in"=w1408) -> ("task out"=w1424:refnum<k21>, "error out"=w1426:errorcluster)  [unwired: 11 in]
        n530 = Index Array(array="AOUT assignment", index #1=0 ("index"), index #2=1 ("index")) -> (element #1=w1395:tag, element #2=w1393:tag)
        n531 = call-poly <vilib>:"DAQmx Create Virtual Channel.vi"("task in"=w1424, "maximum value"=w1423, "minimum value"=w1422, "output terminal configuration"=w1421, "physical channels"=w1395, "units"=w1420, "error in"=w1426) -> ("task out"=w1428:refnum<k21>, "error out"=w1429:errorcluster)  [unwired: 7 in]
        n532 = call-poly <vilib>:"DAQmx Create Virtual Channel.vi"("task in"=w1428, "maximum value"=w1423, "minimum value"=w1422, "physical channels"=w1393, "error in"=w1429) -> ("task out"=w1431:refnum<k21>, "error out"=w1430:errorcluster)  [unwired: 9 in]
        n533 = call <vilib>:"DAQmx Start Task.vi"("task/channels in"=w1431, "error in"=w1430) -> ("task out"=→"AO task out":refnum<k21>, "error out"=w1407:errorcluster)  [unwired: 12 in]
      }
    }
    "error out (USB6210/6218 AOUT)" <- w883
    n534 = case shown="True" w854 {
      frame False {
      }
      frame True {
        n535 = flat-sequence {
          frame #0 {
            n536 = property on="Frontpanel screenshots" class="Bool (strict)"("Val(Sgnl)"=TRUE ("Value (Signaling)")) -> ()  [unwired: 2 in, 2 out]
          }
        }
      }
    }
    n537 = flat-sequence {
      tunnel: w866 -> [w1033]
      tunnel: w869 -> [w1034]
      tunnel: w861 -> [w1286]
      tunnel: w860 -> [w1285]
      frame #0 {
        n538 = stacked-sequence {
          tunnel: w1034 -> [w1039 w1044 w1049 w1054 w1059 w1064 w1069 w1074 w1079 w1084 w1089 w1094 w1099 w1104 w1109 w1114 w1119 w1124 w1129 w1134 w1139 w1144 w1149 w1154 w1159 w1164 w1169 w1174 w1179 w1184 w1189 w1194 w1199 w1204 w1209 w1214 w1219 w1224 w1229 w1234 w1239 w1244 w1249 w1254 w1259 w1264 w1269 w1274 w1279 w1284]
          tunnel: w1033 -> [w1037 w1042 w1047 w1052 w1057 w1062 w1067 w1072 w1077 w1082 w1087 w1092 w1097 w1102 w1107 w1112 w1117 w1122 w1127 w1132 w1137 w1142 w1147 w1152 w1157 w1162 w1167 w1172 w1177 w1182 w1187 w1192 w1197 w1202 w1207 w1212 w1217 w1222 w1227 w1232 w1237 w1242 w1247 w1252 w1257 w1262 w1267 w1272 w1277 w1282]
          frame #0 {
            n539 = Search 1D Array(1D array=w1039, element=T14."T3He1-1" ("SensorLocations")) -> (index of element=w1036:i32)  [unwired: 1 in]
            n540 = Index Array(array=w1037, index=w1036) -> (element=→"T3He1-1":dbl)
          }
          frame #1 {
            n541 = Search 1D Array(1D array=w1044, element=T14."T3He1-2" ("SensorLocations")) -> (index of element=w1041:i32)  [unwired: 1 in]
            n542 = Index Array(array=w1042, index=w1041) -> (element=→"T3He1-2":dbl)
          }
          frame #2 {
            n543 = Search 1D Array(1D array=w1049, element=T14."T3He1-3" ("SensorLocations")) -> (index of element=w1046:i32)  [unwired: 1 in]
            n544 = Index Array(array=w1047, index=w1046) -> (element=→"T3He1-3":dbl)
          }
          frame #3 {
            n545 = Search 1D Array(1D array=w1054, element=T14."T3He1-4" ("SensorLocations")) -> (index of element=w1051:i32)  [unwired: 1 in]
            n546 = Index Array(array=w1052, index=w1051) -> (element=→"T3He1-4":dbl)
          }
          frame #4 {
            n547 = Search 1D Array(1D array=w1059, element=T14."T3He2-1" ("SensorLocations")) -> (index of element=w1056:i32)  [unwired: 1 in]
            n548 = Index Array(array=w1057, index=w1056) -> (element=→"T3He2-1":dbl)
          }
          frame #5 {
            n549 = Search 1D Array(1D array=w1064, element=T14."T3He2-2" ("SensorLocations")) -> (index of element=w1061:i32)  [unwired: 1 in]
            n550 = Index Array(array=w1062, index=w1061) -> (element=→"T3He2-2":dbl)
          }
          frame #6 {
            n551 = Search 1D Array(1D array=w1069, element=T14."T3He3" ("SensorLocations")) -> (index of element=w1066:i32)  [unwired: 1 in]
            n552 = Index Array(array=w1067, index=w1066) -> (element=→"T3He3":dbl)
          }
          frame #7 {
            n553 = Search 1D Array(1D array=w1074, element=T14."T3He4" ("SensorLocations")) -> (index of element=w1071:i32)  [unwired: 1 in]
            n554 = Index Array(array=w1072, index=w1071) -> (element=→"T3He4":dbl)
          }
          frame #8 {
            n555 = Search 1D Array(1D array=w1079, element=T14."T3He5" ("SensorLocations")) -> (index of element=w1076:i32)  [unwired: 1 in]
            n556 = Index Array(array=w1077, index=w1076) -> (element=→"T3He5":dbl)
          }
          frame #9 {
            n557 = Search 1D Array(1D array=w1084, element=T14."T3He6-1" ("SensorLocations")) -> (index of element=w1081:i32)  [unwired: 1 in]
            n558 = Index Array(array=w1082, index=w1081) -> (element=→"T3He6-1" →"T3He6-1/6-2 (HEX1)":dbl)
          }
          frame #10 {
            n559 = Search 1D Array(1D array=w1089, element=T14."T3He6-2" ("SensorLocations")) -> (index of element=w1086:i32)  [unwired: 1 in]
            n560 = Index Array(array=w1087, index=w1086) -> (element=→"T3He6-2" →"T3He6-1/6-2 (3He pot) 2":dbl)
          }
          frame #11 {
            n561 = Search 1D Array(1D array=w1094, element=T14."T3He7-1" ("SensorLocations")) -> (index of element=w1091:i32)  [unwired: 1 in]
            n562 = Index Array(array=w1092, index=w1091) -> (element=→"T3He7-1" →"T3He7-1/7-2 (HEX1)":dbl)
          }
          frame #12 {
            n563 = Search 1D Array(1D array=w1099, element=T14."T3He7-2" ("SensorLocations")) -> (index of element=w1096:i32)  [unwired: 1 in]
            n564 = Index Array(array=w1097, index=w1096) -> (element=→"T3He7-2" →"T3He7-1/6-2 (3He pot) 2":dbl)
          }
          frame #13 {
            n565 = Search 1D Array(1D array=w1104, element=T14."T3He8" ("SensorLocations")) -> (index of element=w1101:i32)  [unwired: 1 in]
            n566 = Index Array(array=w1102, index=w1101) -> (element=→"T3He8":dbl)
          }
          frame #14 {
            n567 = Search 1D Array(1D array=w1109, element=T14."T3He9" ("SensorLocations")) -> (index of element=w1106:i32)  [unwired: 1 in]
            n568 = Index Array(array=w1107, index=w1106) -> (element=→"T3He9":dbl)
          }
          frame #15 {
            n569 = Search 1D Array(1D array=w1114, element=T14."T3He10" ("SensorLocations")) -> (index of element=w1111:i32)  [unwired: 1 in]
            n570 = Index Array(array=w1112, index=w1111) -> (element=→"T3He10":dbl)
          }
          frame #16 {
            n571 = Search 1D Array(1D array=w1119, element=T14."T4He1" ("SensorLocations")) -> (index of element=w1116:i32)  [unwired: 1 in]
            n572 = Index Array(array=w1117, index=w1116) -> (element=→"T4He1" →"T4He1 (4K reservoir )":dbl)
          }
          frame #17 {
            n573 = Search 1D Array(1D array=w1124, element=T14."T4He2-1" ("SensorLocations")) -> (index of element=w1121:i32)  [unwired: 1 in]
            n574 = Index Array(array=w1122, index=w1121) -> (element=→"T4He2-1":dbl)
          }
          frame #18 {
            n575 = Search 1D Array(1D array=w1129, element=T14."T4He2-2" ("SensorLocations")) -> (index of element=w1126:i32)  [unwired: 1 in]
            n576 = Index Array(array=w1127, index=w1126) -> (element=→"T4He2-2":dbl)
          }
          frame #19 {
            n577 = Search 1D Array(1D array=w1134, element=T14."T4He3-1" ("SensorLocations")) -> (index of element=w1131:i32)  [unwired: 1 in]
            n578 = Index Array(array=w1132, index=w1131) -> (element=→"T4He3-1":dbl)
          }
          frame #20 {
            n579 = Search 1D Array(1D array=w1139, element=T14."T4He3-2" ("SensorLocations")) -> (index of element=w1136:i32)  [unwired: 1 in]
            n580 = Index Array(array=w1137, index=w1136) -> (element=→"T4He3-2":dbl)
          }
          frame #21 {
            n581 = Search 1D Array(1D array=w1144, element=T14."T4He3-3" ("SensorLocations")) -> (index of element=w1141:i32)  [unwired: 1 in]
            n582 = Index Array(array=w1142, index=w1141) -> (element=→"T4He3-3":dbl)
          }
          frame #22 {
            n583 = Search 1D Array(1D array=w1149, element=T14."T4He3-4" ("SensorLocations")) -> (index of element=w1146:i32)  [unwired: 1 in]
            n584 = Index Array(array=w1147, index=w1146) -> (element=→"T4He3-4":dbl)
          }
          frame #23 {
            n585 = Search 1D Array(1D array=w1154, element=T14."T4He4" ("SensorLocations")) -> (index of element=w1151:i32)  [unwired: 1 in]
            n586 = Index Array(array=w1152, index=w1151) -> (element=→"T4He4":dbl)
          }
          frame #24 {
            n587 = Search 1D Array(1D array=w1159, element=T14."T4He5" ("SensorLocations")) -> (index of element=w1156:i32)  [unwired: 1 in]
            n588 = Index Array(array=w1157, index=w1156) -> (element=→"T4He5":dbl)
          }
          frame #25 {
            n589 = Search 1D Array(1D array=w1164, element=T14."T4He6" ("SensorLocations")) -> (index of element=w1161:i32)  [unwired: 1 in]
            n590 = Index Array(array=w1162, index=w1161) -> (element=→"T4He6":dbl)
          }
          frame #26 {
            n591 = Search 1D Array(1D array=w1169, element=T14."T4He7" ("SensorLocations")) -> (index of element=w1166:i32)  [unwired: 1 in]
            n592 = Index Array(array=w1167, index=w1166) -> (element=→"T4He7":dbl)
          }
          frame #27 {
            n593 = Search 1D Array(1D array=w1174, element=T14."T4He8" ("SensorLocations")) -> (index of element=w1171:i32)  [unwired: 1 in]
            n594 = Index Array(array=w1172, index=w1171) -> (element=→"T4He8":dbl)
          }
          frame #28 {
            n595 = Search 1D Array(1D array=w1179, element=T14."T4He9" ("SensorLocations")) -> (index of element=w1176:i32)  [unwired: 1 in]
            n596 = Index Array(array=w1177, index=w1176) -> (element=→"T4He9":dbl)
          }
          frame #29 {
            n597 = Search 1D Array(1D array=w1184, element=T14."T4He10" ("SensorLocations")) -> (index of element=w1181:i32)  [unwired: 1 in]
            n598 = Index Array(array=w1182, index=w1181) -> (element=→"T4He10":dbl)
          }
          frame #30 {
            n599 = Search 1D Array(1D array=w1189, element=T14."T1K1" ("SensorLocations")) -> (index of element=w1186:i32)  [unwired: 1 in]
            n600 = Index Array(array=w1187, index=w1186) -> (element=→"T1K1":dbl)
          }
          frame #31 {
            n601 = Search 1D Array(1D array=w1194, element=T14."T1K2" ("SensorLocations")) -> (index of element=w1191:i32)  [unwired: 1 in]
            n602 = Index Array(array=w1192, index=w1191) -> (element=→"T1K2":dbl)
          }
          frame #32 {
            n603 = Search 1D Array(1D array=w1199, element=T14."T1K3-1" ("SensorLocations")) -> (index of element=w1196:i32)  [unwired: 1 in]
            n604 = Index Array(array=w1197, index=w1196) -> (element=→"T1K3-1" →"T1K3-1/3-2 (1K pot)":dbl)
          }
          frame #33 {
            n605 = Search 1D Array(1D array=w1204, element=T14."T1K3-2" ("SensorLocations")) -> (index of element=w1201:i32)  [unwired: 1 in]
            n606 = Index Array(array=w1202, index=w1201) -> (element=→"T1K3-2" →"T1K3-1/3-2 (1K pot) 2":dbl)
          }
          frame #34 {
            n607 = Search 1D Array(1D array=w1209, element=T14."T1K4" ("SensorLocations")) -> (index of element=w1206:i32)  [unwired: 1 in]
            n608 = Index Array(array=w1207, index=w1206) -> (element=→"T1K4":dbl)
          }
          frame #35 {
            n609 = Search 1D Array(1D array=w1214, element=T14."T1K5" ("SensorLocations")) -> (index of element=w1211:i32)  [unwired: 1 in]
            n610 = Index Array(array=w1212, index=w1211) -> (element=→"T1K5":dbl)
          }
          frame #36 {
            n611 = Search 1D Array(1D array=w1219, element=T14."T1K6" ("SensorLocations")) -> (index of element=w1216:i32)  [unwired: 1 in]
            n612 = Index Array(array=w1217, index=w1216) -> (element=→"T1K6":dbl)
          }
          frame #37 {
            n613 = Search 1D Array(1D array=w1224, element=T14."TIP1" ("SensorLocations")) -> (index of element=w1221:i32)  [unwired: 1 in]
            n614 = Index Array(array=w1222, index=w1221) -> (element=→"TIP1":dbl)
          }
          frame #38 {
            n615 = Search 1D Array(1D array=w1229, element=T14."TIP2" ("SensorLocations")) -> (index of element=w1226:i32)  [unwired: 1 in]
            n616 = Index Array(array=w1227, index=w1226) -> (element=→"TIP2":dbl)
          }
          frame #39 {
            n617 = Search 1D Array(1D array=w1234, element=T14."TIP3" ("SensorLocations")) -> (index of element=w1231:i32)  [unwired: 1 in]
            n618 = Index Array(array=w1232, index=w1231) -> (element=→"TIP3":dbl)
          }
          frame #40 {
            n619 = Search 1D Array(1D array=w1239, element=T14."TIP4" ("SensorLocations")) -> (index of element=w1236:i32)  [unwired: 1 in]
            n620 = Index Array(array=w1237, index=w1236) -> (element=→"TIP4":dbl)
          }
          frame #41 {
            n621 = Search 1D Array(1D array=w1244, element=T14."TIP5" ("SensorLocations")) -> (index of element=w1241:i32)  [unwired: 1 in]
            n622 = Index Array(array=w1242, index=w1241) -> (element=→"TIP5":dbl)
          }
          frame #42 {
            n623 = Search 1D Array(1D array=w1249, element=T14."TIP6" ("SensorLocations")) -> (index of element=w1246:i32)  [unwired: 1 in]
            n624 = Index Array(array=w1247, index=w1246) -> (element=→"TIP6":dbl)
          }
          frame #43 {
            n625 = Search 1D Array(1D array=w1254, element=T14."TIP7" ("SensorLocations")) -> (index of element=w1251:i32)  [unwired: 1 in]
            n626 = Index Array(array=w1252, index=w1251) -> (element=→"TIP7":dbl)
          }
          frame #44 {
            n627 = Search 1D Array(1D array=w1259, element=T14."TTH1" ("SensorLocations")) -> (index of element=w1256:i32)  [unwired: 1 in]
            n628 = Index Array(array=w1257, index=w1256) -> (element=→"TTH1":dbl)
          }
          frame #45 {
            n629 = Search 1D Array(1D array=w1264, element=T14."TTH2" ("SensorLocations")) -> (index of element=w1261:i32)  [unwired: 1 in]
            n630 = Index Array(array=w1262, index=w1261) -> (element=→"TTH2":dbl)
          }
          frame #46 {
            n631 = Search 1D Array(1D array=w1269, element=T14."TTH3" ("SensorLocations")) -> (index of element=w1266:i32)  [unwired: 1 in]
            n632 = Index Array(array=w1267, index=w1266) -> (element=→"TTH3":dbl)
          }
          frame #47 {
            n633 = Search 1D Array(1D array=w1274, element=T14."TTH4" ("SensorLocations")) -> (index of element=w1271:i32)  [unwired: 1 in]
            n634 = Index Array(array=w1272, index=w1271) -> (element=→"TTH4":dbl)
          }
          frame #48 {
            n635 = Search 1D Array(1D array=w1279, element="SensorLocation 1") -> (index of element=w1276:i32)  [unwired: 1 in]
            n636 = Index Array(array=w1277, index=w1276) -> (element=→"Temperature 1":dbl)
          }
          frame #49 {
            n637 = Search 1D Array(1D array=w1284, element="SensorLocation 2") -> (index of element=w1281:i32)  [unwired: 1 in]
            n638 = Index Array(array=w1282, index=w1281) -> (element=→"Temperature 2":dbl)
          }
        }
      }
      frame #1 {
        n639 = stacked-sequence {
          tunnel: w1286 -> [w1291 w1296 w1301 w1306 w1311 w1316 w1321 w1326 w1331 w1336 w1341 w1346 w1351 w1356 w1361 w1366 w1371 w1376 w1381]
          tunnel: w1285 -> [w1288 w1294 w1300 w1305 w1310 w1314 w1319 w1324 w1329 w1334 w1339 w1344 w1348 w1353 w1358 w1363 w1368 w1373 _]
          tunnel: w1285 -> [_ _ _ _ _ _ _ _ _ _ _ _ _ _ _ _ _ _ w1379]
          frame #0 {
            n640 = Search 1D Array(1D array=w1291, element="Insulation vacuum") -> (index of element=w1289:i32)  [unwired: 1 in]
            n641 = Index Array(array=w1288, index=w1289) -> (element=→"P_ins" →"P (insulation)":dbl)
          }
          frame #1 {
            n642 = Search 1D Array(1D array=w1296, element="4K reservoir pressure") -> (index of element=w1293:i32)  [unwired: 1 in]
            n643 = Index Array(array=w1294, index=w1293) -> (element=→"P_4Kres" →"P (4K reservoir)":dbl)